vi "Dresden R2R Sputter 03.02.2018 IY24.vi"() -> ()   [LabVIEW 2009] (continued)
                                }
                                }
                                }
                                }
                                frame #4 {
                                n32415 = local read "R Cmb Ch2 Step5 Coating Power Active"() -> (w37013:bool)
                                n32416 = case shown="True" w37013 {
                                frame #0 {
                                }
                                frame #1 {
                                n32417 = stacked-sequence {
                                frame #0 {
                                n32418 = local read "Semi"() -> (w37014:bool)
                                n32419 = case shown="False" w37014 {
                                frame #0 {
                                n32420 = local read "R Cmb Ch3 Step5 Coating Power"() -> (w37016:dbl)
                                n32421 = Wait (ms)(milliseconds to wait=u32 200) -> ()  [unwired: 1 out]
                                n32422 = local write "Set DC Power       : 2"(w37016) -> ()
                                }
                                frame #1 {
                                }
                                }
                                }
                                frame #1 {
                                n32423 = local read "Semi"() -> (w37017:bool)
                                n32424 = case shown="False" w37017 {
                                frame #0 {
                                n32425 = local write "Dc_auto_set"(TRUE ("Dc_auto_set")) -> ()
                                }
                                frame #1 {
                                }
                                }
                                }
                                frame #2 {
                                n32426 = while {
                                stop <- w37023 stop-if-true
                                n32427 = local read "R Cmb Interval length"() -> (w37022:dbl)
                                n32428 = local read "Actual Length"() -> (w37026:dbl)
                                n32429 = Multiply(x=w37022, y=5.0) -> (x*y=w37020:dbl)
                                n32430 = Greater Or Equal?(x=w37026, y=w37020) -> (x >= y?=w37025:bool)
                                n32431 = local read "Semi"() -> (w37024:bool)
                                n32432 = Or(x=w37025, y=w37024) -> (x .or. y?=w37023:bool)
                                n32433 = Wait Until Next ms Multiple(millisecond multiple=u32 300) -> ()  [unwired: 1 out]
                                }
                                }
                                }
                                }
                                }
                                }
                                }
                                }
                                frame #1 {
                                }
                                }
                                }
                                frame #13 {
                                n32434 = local read "Semi"() -> (w37027:bool)
                                n32435 = case shown="False" w37027 {
                                frame #0 {
                                n32436 = local write "SDC1 13b"(TRUE ("SDC1 13b")) -> ()
                                n32437 = Wait (ms)(milliseconds to wait=u32 1000) -> ()  [unwired: 1 out]
                                }
                                frame #1 {
                                }
                                }
                                }
                                }
                                }
                                frame #13 {
                                # "CLOSE DC"
                                n32438 = local read "Semi"() -> (w37030:bool)
                                n32439 = case shown="False" w37030 {
                                frame #0 {
                                n32440 = stacked-sequence {
                                frame #0 {
                                n32441 = local read "Semi"() -> (w37031:bool)
                                n32442 = case shown="False" w37031 {
                                frame #0 {
                                n32443 = local write "Dc_auto_off"(TRUE ("Dc_auto_off")) -> ()
                                }
                                frame #1 {
                                }
                                }
                                }
                                frame #1 {
                                n32444 = local read "Semi"() -> (w37033:bool)
                                n32445 = case shown="False" w37033 {
                                frame #0 {
                                n32446 = Wait (ms)(milliseconds to wait=u32 1000) -> ()  [unwired: 1 out]
                                }
                                frame #1 {
                                }
                                }
                                }
                                frame #2 {
                                n32447 = local read "Semi"() -> (w37035:bool)
                                n32448 = case shown="False" w37035 {
                                frame #0 {
                                n32449 = local write "Dc_auto_set_zero"(TRUE ("Dc_auto_set")) -> ()
                                }
                                frame #1 {
                                }
                                }
                                }
                                frame #3 {
                                n32450 = local read "Semi"() -> (w37037:bool)
                                n32451 = case shown="False" w37037 {
                                frame #0 {
                                n32452 = Wait (ms)(milliseconds to wait=u32 1000) -> ()  [unwired: 1 out]
                                }
                                frame #1 {
                                }
                                }
                                }
                                frame #4 {
                                n32453 = local read "Semi"() -> (w37039:bool)
                                n32454 = case shown="False" w37039 {
                                frame #0 {
                                n32455 = while {
                                i -> [w37051]
                                stop <- w37040 stop-if-true
                                n32456 = Greater?(x=w37051, y=600) -> (0:w37050:bool)
                                n32457 = case shown="True" w37050 {
                                frame #0 {
                                }
                                frame #1 {
                                n32458 = local write "Semi"(TRUE ("Semi")) -> ()
                                n32459 = local write "Error Message"("Sputter Process cancelled.\nPlease Check DC connections." ("Error Message")) -> ()
                                }
                                }
                                n32460 = local read "Actual DC Power : 2"() -> (w37045:dbl)
                                n32461 = local read "Actual DC Volt2"() -> (w37044:dbl)
                                n32462 = Less?(x=w37045, y=10.0) -> (x < y?=w37048:bool)
                                n32463 = Less?(x=w37044, y=20.0) -> (x < y?=w37049:bool)
                                n32464 = And(x=w37048, y=w37049) -> (x .and. y?=w37042:bool)
                                n32465 = local read "Semi"() -> (w37041:bool)
                                n32466 = Wait Until Next ms Multiple(millisecond multiple=u32 500) -> ()  [unwired: 1 out]
                                n32467 = Compound Arithmetic op=OR(w37042, w37041) -> (w37040:bool)
                                }
                                }
                                frame #1 {
                                }
                                }
                                }
                                frame #5 {
                                n32468 = local read "Semi"() -> (w37055:bool)
                                n32469 = case shown="False" w37055 {
                                frame #0 {
                                n32470 = while {
                                i -> [w37061]
                                stop <- w37056 stop-if-true
                                n32471 = Greater?(x=w37061, y=50) -> (0:w37060:bool)
                                n32472 = case shown="True" w37060 {
                                frame #0 {
                                }
                                frame #1 {
                                n32473 = local write "Semi"(TRUE ("Semi")) -> ()
                                n32474 = local write "Error Message"("Sputter Process cancelled.\nPlease Check DCPS-SW2." ("Error Message")) -> ()
                                }
                                }
                                n32475 = local read "Cnt_Dcps_sw2_di"() -> (w37059:bool)
                                n32476 = case shown="True" w37059 {
                                tunnel: [TRUE ("Cnt_Dcps_sw1_do") FALSE ("Cnt_Dcps_sw1_do")] -> w37058
                                frame #0 {
                                }
                                frame #1 {
                                n32477 = local write "Cnt_Dcps_sw2_do"(FALSE ("Cnt_Dcps_sw1_do")) -> ()
                                n32478 = Wait Until Next ms Multiple(millisecond multiple=u32 500) -> ()  [unwired: 1 out]
                                }
                                }
                                n32479 = local read "Semi"() -> (w37057:bool)
                                n32480 = Or(x=w37058, y=w37057) -> (x .or. y?=w37056:bool)
                                }
                                }
                                frame #1 {
                                }
                                }
                                }
                                frame #6 {
                                n32481 = local read "Semi"() -> (w37069:bool)
                                n32482 = case shown="False" w37069 {
                                frame #0 {
                                n32483 = Wait (ms)(milliseconds to wait=u32 1000) -> ()  [unwired: 1 out]
                                n32484 = local write "SDC1 25"(TRUE ("SDC1 25")) -> ()
                                }
                                frame #1 {
                                }
                                }
                                }
                                }
                                }
                                frame #1 {
                                }
                                }
                                }
                                frame #14 {
                                # "PC-BV OPEN"
                                n32485 = stacked-sequence {
                                frame #0 {
                                n32486 = local read "Semi"() -> (w37072:bool)
                                n32487 = case shown="False" w37072 {
                                frame #0 {
                                n32488 = stacked-sequence {
                                frame #0 {
                                n32489 = local read "Semi"() -> (w37073:bool)
                                n32490 = case shown="False" w37073 {
                                frame #0 {
                                n32491 = local write "Pc_bv3_auto_open"(TRUE ("Tp1_auto_start")) -> ()
                                }
                                frame #1 {
                                }
                                }
                                }
                                frame #1 {
                                n32492 = local read "Semi"() -> (w37075:bool)
                                n32493 = case shown="False" w37075 {
                                frame #0 {
                                n32494 = Wait (ms)(milliseconds to wait=u32 1000) -> ()  [unwired: 1 out]
                                }
                                frame #1 {
                                }
                                }
                                }
                                frame #2 {
                                n32495 = local read "Semi"() -> (w37077:bool)
                                n32496 = case shown="False" w37077 {
                                frame #0 {
                                n32497 = while {
                                i -> [w37083]
                                stop <- w37079 stop-if-true
                                n32498 = local read "Pc_bv_opened_ch3"() -> (w37081:bool)
                                n32499 = Greater?(x=w37083, y=120) -> (0:w37082:bool)
                                n32500 = local read "Semi"() -> (w37080:bool)
                                n32501 = Compound Arithmetic op=OR(w37080, w37081, w37082) -> (w37079:bool)
                                n32502 = Wait (ms)(milliseconds to wait=u32 500) -> ()  [unwired: 1 out]
                                }
                                }
                                frame #1 {
                                }
                                }
                                }
                                frame #3 {
                                n32503 = local read "Semi"() -> (w37085:bool)
                                n32504 = case shown="False" w37085 {
                                frame #0 {
                                n32505 = local read "Pc_bv_opened_ch3"() -> (w37086:bool)
                                n32506 = case shown="False" w37086 {
                                frame #0 {
                                n32507 = local write "Pc_bv3_auto_open"(TRUE ("Pc_bv1_auto_open")) -> ()
                                }
                                frame #1 {
                                }
                                }
                                }
                                frame #1 {
                                }
                                }
                                }
                                frame #4 {
                                n32508 = local read "Semi"() -> (w37088:bool)
                                n32509 = case shown="False" w37088 {
                                frame #0 {
                                n32510 = local read "Pc_bv_opened_ch3"() -> (w37089:bool)
                                n32511 = case shown="False" w37089 {
                                frame #0 {
                                n32512 = Wait (ms)(milliseconds to wait=u32 1000) -> ()  [unwired: 1 out]
                                }
                                frame #1 {
                                }
                                }
                                }
                                frame #1 {
                                }
                                }
                                }
                                frame #5 {
                                n32513 = local read "Semi"() -> (w37091:bool)
                                n32514 = case shown="False" w37091 {
                                frame #0 {
                                n32515 = while {
                                i -> [w37097]
                                stop <- w37093 stop-if-true
                                n32516 = local read "Pc_bv_opened_ch3"() -> (w37095:bool)
                                n32517 = Greater?(x=w37097, y=120) -> (0:w37096:bool)
                                n32518 = local read "Semi"() -> (w37094:bool)
                                n32519 = Compound Arithmetic op=OR(w37094, w37095, w37096) -> (w37093:bool)
                                n32520 = Wait (ms)(milliseconds to wait=u32 500) -> ()  [unwired: 1 out]
                                }
                                }
                                frame #1 {
                                }
                                }
                                }
                                frame #6 {
                                n32521 = local read "Semi"() -> (w37099:bool)
                                n32522 = case shown="False" w37099 {
                                frame #0 {
                                n32523 = local read "Pc_bv_opened_ch3"() -> (w37100:bool)
                                n32524 = case shown="False" w37100 {
                                frame #0 {
                                n32525 = local write "Error Message"("Start up process  cancelled\nbecause  PC-BV not opened.\nPlease check PC-BV1 connections." ("Error Message")) -> ()
                                n32526 = Wait (ms)(milliseconds to wait=u32 1000) -> ()  [unwired: 1 out]
                                }
                                frame #1 {
                                }
                                }
                                }
                                frame #1 {
                                }
                                }
                                }
                                }
                                }
                                frame #1 {
                                }
                                }
                                }
                                frame #1 {
                                n32527 = local read "Semi"() -> (w37103:bool)
                                n32528 = case shown="False" w37103 {
                                frame #0 {
                                n32529 = Wait (ms)(milliseconds to wait=u32 1000) -> ()  [unwired: 1 out]
                                n32530 = local write "SDC1 28"(TRUE ("SDC1 28")) -> ()
                                }
                                frame #1 {
                                }
                                }
                                }
                                }
                                }
                                frame #15 {
                                # "set ar zero"
                                n32531 = stacked-sequence {
                                frame #0 {
                                n32532 = local read "Semi"() -> (w37106:bool)
                                n32533 = case shown="False" w37106 {
                                frame #0 {
                                n32534 = stacked-sequence {
                                frame #0 {
                                n32535 = local read "Semi"() -> (w37107:bool)
                                n32536 = case shown="False" w37107 {
                                frame #0 {
                                n32537 = local write "Ar_auto_set_zero_ch3"(TRUE ("Ar_auto_set_zero_ch1")) -> ()
                                }
                                frame #1 {
                                }
                                }
                                }
                                frame #1 {
                                n32538 = local read "Semi"() -> (w37109:bool)
                                n32539 = case shown="False" w37109 {
                                frame #0 {
                                n32540 = while {
                                i -> [w37112]
                                stop <- w37111 stop-if-true
                                n32541 = Greater?(x=w37112, y=150) -> (0:w37111:bool)
                                n32542 = local read "Semi"() -> (w37110:bool)
                                n32543 = case shown="False" w37110 {
                                tunnel: [FALSE TRUE] -> _
                                frame #0 {
                                n32544 = Wait Until Next ms Multiple(millisecond multiple=u32 200) -> ()  [unwired: 1 out]
                                }
                                frame #1 {
                                }
                                }
                                }
                                }
                                frame #1 {
                                }
                                }
                                }
                                frame #2 {
                                n32545 = local read "Semi"() -> (w37117:bool)
                                n32546 = case shown="False" w37117 {
                                frame #0 {
                                n32547 = local read "Ar_sccm_act 2"() -> (w37118:dbl)
                                n32548 = Less?(x=w37118, y=1) -> (x < y?=w37119:bool)
                                n32549 = case shown="False" w37119 {
                                frame #0 {
                                n32550 = local write "Ar_auto_set_zero_ch3"(TRUE ("Ar_auto_set_zero_ch1")) -> ()
                                }
                                frame #1 {
                                }
                                }
                                }
                                frame #1 {
                                }
                                }
                                }
                                frame #3 {
                                n32551 = local read "Semi"() -> (w37122:bool)
                                n32552 = case shown="False" w37122 {
                                frame #0 {
                                n32553 = local read "Ar_sccm_act 2"() -> (w37123:dbl)
                                n32554 = Less?(x=w37123, y=1) -> (x < y?=w37124:bool)
                                n32555 = case shown="False" w37124 {
                                frame #0 {
                                n32556 = while {
                                i -> [w37130]
                                stop <- w37127 stop-if-true
                                n32557 = Greater?(x=w37130, y=150) -> (0:w37128:bool)
                                n32558 = local read "Semi"() -> (w37126:bool)
                                n32559 = case shown="True" w37126 {
                                tunnel: [FALSE FALSE] -> w37129
                                frame #0 {
                                }
                                frame #1 {
                                n32560 = Wait Until Next ms Multiple(millisecond multiple=u32 200) -> ()  [unwired: 1 out]
                                }
                                }
                                n32561 = Or(x=w37129, y=w37128) -> (x .or. y?=w37127:bool)
                                }
                                }
                                frame #1 {
                                }
                                }
                                }
                                frame #1 {
                                }
                                }
                                }
                                frame #4 {
                                n32562 = local read "Semi"() -> (w37135:bool)
                                n32563 = case shown="False" w37135 {
                                frame #0 {
                                n32564 = Wait (ms)(milliseconds to wait=u32 1000) -> ()  [unwired: 1 out]
                                }
                                frame #1 {
                                }
                                }
                                }
                                }
                                }
                                frame #1 {
                                }
                                }
                                }
                                frame #1 {
                                n32565 = local read "Semi"() -> (w37137:bool)
                                n32566 = case shown="False" w37137 {
                                frame #0 {
                                n32567 = local write "SDC1 26"(TRUE ("SDC1 26")) -> ()
                                n32568 = Wait (ms)(milliseconds to wait=u32 1000) -> ()  [unwired: 1 out]
                                }
                                frame #1 {
                                }
                                }
                                }
                                }
                                }
                                frame #16 {
                                # "sov-ar close"
                                n32569 = stacked-sequence {
                                frame #0 {
                                n32570 = local read "Semi"() -> (w37140:bool)
                                n32571 = case shown="False" w37140 {
                                frame #0 {
                                n32572 = while {
                                i -> [w37146]
                                stop <- w37141 stop-if-true
                                n32573 = Greater?(x=w37146, y=50) -> (0:w37145:bool)
                                n32574 = case shown="True" w37145 {
                                frame #0 {
                                }
                                frame #1 {
                                n32575 = local write "Semi"(TRUE ("Semi")) -> ()
                                n32576 = local write "Error Message"("Coating Process  \nwas cancelled.\nPlease check \nSOV-Ar connection." ("Error Message")) -> ()
                                }
                                }
                                n32577 = local read "Ch3_Sov_Ar_di"() -> (w37144:bool)
                                n32578 = case shown="True" w37144 {
                                tunnel: [TRUE FALSE] -> w37143
                                frame #0 {
                                }
                                frame #1 {
                                n32579 = local write "Ch3_Sov_Ar_do"(FALSE ("Ch1_WFC_do")) -> ()
                                n32580 = Wait Until Next ms Multiple(millisecond multiple=u32 200) -> ()  [unwired: 1 out]
                                }
                                }
                                n32581 = local read "Semi"() -> (w37142:bool)
                                n32582 = Or(x=w37143, y=w37142) -> (x .or. y?=w37141:bool)
                                }
                                }
                                frame #1 {
                                }
                                }
                                }
                                frame #1 {
                                n32583 = local read "Semi"() -> (w37154:bool)
                                n32584 = case shown="False" w37154 {
                                frame #0 {
                                n32585 = local write "SDC1 27"(TRUE ("SDC1 27")) -> ()
                                n32586 = Wait (ms)(milliseconds to wait=u32 1000) -> ()  [unwired: 1 out]
                                }
                                frame #1 {
                                }
                                }
                                }
                                }
                                }
                                frame #17 {
                                # "CC OPEN"
                                n32587 = stacked-sequence {
                                frame #0 {
                                n32588 = local read "Semi"() -> (w37157:bool)
                                n32589 = case shown="False" w37157 {
                                frame #0 {
                                n32590 = while {
                                i -> [w37163]
                                stop <- w37158 stop-if-true
                                n32591 = Greater?(x=w37163, y=50) -> (0:w37162:bool)
                                n32592 = case shown="True" w37162 {
                                frame #0 {
                                }
                                frame #1 {
                                n32593 = local write "Semi"(TRUE ("Semi")) -> ()
                                n32594 = local write "Error Message"("Coating Process  \nwas cancelled.\nPlease check \nBG-BV connection." ("Error Message")) -> ()
                                }
                                }
                                n32595 = local read "Ch3_Cc_on_off_di"() -> (w37161:bool)
                                n32596 = case shown="False" w37161 {
                                tunnel: [FALSE TRUE] -> w37160
                                frame #0 {
                                n32597 = local write "Ch3_Cc_on_off_do"(TRUE ("Ch1_WFC_do")) -> ()
                                n32598 = Wait Until Next ms Multiple(millisecond multiple=u32 200) -> ()  [unwired: 1 out]
                                }
                                frame #1 {
                                }
                                }
                                n32599 = local read "Semi"() -> (w37159:bool)
                                n32600 = Or(x=w37160, y=w37159) -> (x .or. y?=w37158:bool)
                                }
                                }
                                frame #1 {
                                }
                                }
                                }
                                frame #1 {
                                n32601 = local read "Semi"() -> (w37171:bool)
                                n32602 = case shown="False" w37171 {
                                frame #0 {
                                n32603 = while {
                                i -> [w37176]
                                stop <- w37174 stop-if-true
                                n32604 = Greater?(x=w37176, y=30) -> (0:w37172:bool)
                                n32605 = Wait Until Next ms Multiple(millisecond multiple=u32 1000) -> ()  [unwired: 1 out]
                                n32606 = local read "Semi"() -> (w37175:bool)
                                n32607 = Or(x=w37172, y=w37175) -> (x .or. y?=w37174:bool)
                                }
                                }
                                frame #1 {
                                }
                                }
                                }
                                frame #2 {
                                n32608 = local read "Semi"() -> (w37178:bool)
                                n32609 = case shown="False" w37178 {
                                frame #0 {
                                n32610 = local write "SDC1 27b"(TRUE ("SDC1 3")) -> ()
                                n32611 = Wait (ms)(milliseconds to wait=u32 1000) -> ()  [unwired: 1 out]
                                }
                                frame #1 {
                                }
                                }
                                }
                                }
                                }
                                frame #18 {
                                # "CHECK CHAMBER PRESSURE"
                                n32612 = stacked-sequence {
                                frame #0 {
                                n32613 = local read "Semi"() -> (w37181:bool)
                                n32614 = case shown="False" w37181 {
                                frame #0 {
                                n32615 = while {
                                i -> [w37189]
                                stop <- w37183 stop-if-true
                                n32616 = Greater?(x=w37189, y=300) -> (0:w37188:bool)
                                n32617 = case shown="True" w37188 {
                                frame #0 {
                                }
                                frame #1 {
                                n32618 = local write "Semi"(TRUE ("Semi")) -> ()
                                n32619 = local write "Error Message"("Coating Process cancelled.\nPlease check chamber \nconnections." ("Error Message")) -> ()
                                }
                                }
                                n32620 = local read "Ch_CC_press_ch3 2"() -> (w37182:dbl)
                                n32621 = Greater Or Equal?(x=w37182, y=5e-05 ("CHAMBER PRESSURE 6")) -> (x >= y?=w37186:bool)
                                n32622 = case shown="True" w37186 {
                                tunnel: [TRUE FALSE] -> w37185
                                frame #0 {
                                }
                                frame #1 {
                                n32623 = Wait Until Next ms Multiple(millisecond multiple=u32 200) -> ()  [unwired: 1 out]
                                }
                                }
                                n32624 = local read "Semi"() -> (w37184:bool)
                                n32625 = Or(x=w37185, y=w37184) -> (x .or. y?=w37183:bool)
                                }
                                }
                                frame #1 {
                                }
                                }
                                }
                                frame #1 {
                                n32626 = local read "Semi"() -> (w37196:bool)
                                n32627 = case shown="False" w37196 {
                                frame #0 {
                                n32628 = Wait (ms)(milliseconds to wait=u32 1000) -> ()  [unwired: 1 out]
                                n32629 = local write "SDC1 27c"(TRUE ("SDC1 10")) -> ()
                                }
                                frame #1 {
                                }
                                }
                                }
                                }
                                }
                                frame #19 {
                                # "encoder info  add to other web selection"
                                n32630 = stacked-sequence {
                                frame #0 {
                                n32631 = local read "Semi"() -> (w37199:bool)
                                n32632 = case shown="False" w37199 {
                                frame #0 {
                                # "TC -ROLL"
                                n32633 = local read "Semi"() -> (w37200:bool)
                                n32634 = case shown="False" w37200 {
                                frame #0 {
                                n32635 = stacked-sequence {
                                frame #0 {
                                n32636 = local read "R Web speed(cm/min)"() -> (w37203:dbl)
                                n32637 = local read "R Maximum diameter"() -> (w37201:dbl)
                                n32638 = local read "R Web thicness"() -> (w37202:dbl)
                                n32639 = local write "Change_Max Diameter"(w37201) -> ()
                                n32640 = Wait (ms)(milliseconds to wait=u32 100) -> ()  [unwired: 1 out]
                                n32641 = local write "Web Thickness"(w37202) -> ()
                                n32642 = local write "Web Speed"(w37203) -> ()
                                }
                                frame #1 {
                                n32643 = local write "Calculate 3"(TRUE ("Calculate 3")) -> ()
                                }
                                frame #2 {
                                n32644 = local read "R Cmb Ch2 Step1 Coating Power Active"() -> (w37207:bool)
                                n32645 = local read "R Cmb Ch2 Step2 Coating Power Active"() -> (w37208:bool)
                                n32646 = local read "R Cmb Ch2 Step3 Coating Power Active"() -> (w37209:bool)
                                n32647 = local read "R Cmb Ch2 Step4 Coating Power Active"() -> (w37210:bool)
                                n32648 = local read "R Cmb Ch2 Step5 Coating Power Active"() -> (w37211:bool)
                                n32649 = Boolean To (0,1)(Boolean=w37207) -> (0, 1=w37212:i16)
                                n32650 = Boolean To (0,1)(Boolean=w37208) -> (0, 1=w37213:i16)
                                n32651 = Boolean To (0,1)(Boolean=w37209) -> (0, 1=w37214:i16)
                                n32652 = Boolean To (0,1)(Boolean=w37210) -> (0, 1=w37215:i16)
                                n32653 = Boolean To (0,1)(Boolean=w37211) -> (0, 1=w37216:i16)
                                n32654 = Compound Arithmetic op=ADD(w37212, w37213, w37214, w37215, w37216) -> (w37218:i16)
                                n32655 = local read "R Cmb Interval length"() -> (w37217:dbl)
                                n32656 = Wait (ms)(milliseconds to wait=u32 200) -> ()  [unwired: 1 out]
                                n32657 = Multiply(x=w37217, y=w37218) -> (x*y=w37219:dbl)
                                n32658 = local write "Total length"(w37219) -> ()
                                }
                                frame #3 {
                                n32659 = Wait (ms)(milliseconds to wait=u32 1000) -> ()  [unwired: 1 out]
                                }
                                frame #4 {
                                n32660 = local read "Change_Max Diameter"() -> (w37222:dbl)
                                n32661 = Wait (ms)(milliseconds to wait=u32 200) -> ()  [unwired: 1 out]
                                n32662 = local write "Initial Min Diameter"(w37222) -> ()
                                }
                                frame #5 {
                                n32663 = local write "Calculate 2"(TRUE ("Calculate_auto")) -> ()
                                }
                                frame #6 {
                                n32664 = local write "Roll_side_select"(enum32{"Left to Right", "Right to Left"}."Right to Left" ("Roll_side_select")) -> ()
                                }
                                frame #7 {
                                n32665 = Wait (ms)(milliseconds to wait=u32 100) -> ()  [unwired: 1 out]
                                n32666 = local write "Parameters_auto_set"(TRUE ("Parameters_auto_set")) -> ()
                                }
                                frame #8 {
                                n32667 = while {
                                i -> [w37231]
                                stop <- w37227 stop-if-true
                                n32668 = Wait Until Next ms Multiple(millisecond multiple=u32 300) -> ()  [unwired: 1 out]
                                n32669 = Greater?(x=w37231, y=100) -> (0:w37228:bool)
                                n32670 = local read "Parameters_auto_set"() -> (w37232:bool)
                                n32671 = case shown="False" w37232 {
                                tunnel: [TRUE FALSE] -> w37229
                                frame #0 {
                                }
                                frame #1 {
                                }
                                }
                                n32672 = Or(x=w37229, y=w37228) -> (x .or. y?=w37227:bool)
                                }
                                }
                                frame #9 {
                                n32673 = local read "R Tension Value"() -> (w37236:dbl)
                                n32674 = Wait (ms)(milliseconds to wait=u32 200) -> ()  [unwired: 1 out]
                                n32675 = local write "TC2_set_value"(w37236) -> ()
                                }
                                frame #10 {
                                n32676 = local write "TC2_auto_set"(TRUE ("TC1_auto_set")) -> ()
                                }
                                frame #11 {
                                w37239 = u16 2 items=["1", "2", "3", "4"] ("Target Chamber Sensor")
                                n32677 = local write "Target Chamber Sensor"(w37239) -> ()
                                }
                                frame #12 {
                                n32678 = local read "Total length"() -> (w37240:dbl)
                                n32679 = local write "Region"(w37240) -> ()
                                }
                                frame #13 {
                                n32680 = local read "Semi"() -> (w37241:bool)
                                n32681 = case shown="False" w37241 {
                                frame #0 {
                                n32682 = local write "Start_roll"(TRUE ("Start_roll")) -> ()
                                n32683 = Wait (ms)(milliseconds to wait=u32 300) -> ()  [unwired: 1 out]
                                }
                                frame #1 {
                                }
                                }
                                }
                                frame #14 {
                                n32684 = local read "Semi"() -> (w37244:bool)
                                n32685 = case shown="False" w37244 {
                                frame #0 {
                                n32686 = while {
                                stop <- w37248 stop-if-true
                                n32687 = Wait Until Next ms Multiple(millisecond multiple=u32 200 ("milliseconds to wait")) -> ()  [unwired: 1 out]
                                n32688 = local read "Start_roll"() -> (w37246:bool)
                                n32689 = Not(x=w37246) -> (.not. x?=w37245:bool)
                                n32690 = local read "Semi"() -> (w37249:bool)
                                n32691 = Or(x=w37245, y=w37249) -> (x .or. y?=w37248:bool)
                                }
                                }
                                frame #1 {
                                }
                                }
                                }
                                }
                                }
                                frame #1 {
                                }
                                }
                                }
                                frame #1 {
                                }
                                }
                                }
                                frame #1 {
                                n32692 = local read "Semi"() -> (w37250:bool)
                                n32693 = case shown="False" w37250 {
                                frame #0 {
                                n32694 = Wait (ms)(milliseconds to wait=u32 1000) -> ()  [unwired: 1 out]
                                n32695 = local write "SDC1 29"(TRUE ("SDC1 29")) -> ()
                                }
                                frame #1 {
                                }
                                }
                                }
                                }
                                }
                                frame #20 {
                                n32696 = local read "Semi"() -> (w37253:bool)
                                n32697 = case shown="False" w37253 {
                                frame #0 {
                                n32698 = Wait (ms)(milliseconds to wait=u32 2500) -> ()  [unwired: 1 out]
                                n32699 = local write "SDC1 30"(TRUE ("SDC1 30")) -> ()
                                n32700 = local write "Cnt_Do_Buzzer"(TRUE ("SDC1 30")) -> ()
                                }
                                frame #1 {
                                }
                                }
                                }
                                frame #21 {
                                n32701 = local read "Semi"() -> (w37257:bool)
                                n32702 = case shown="False" w37257 {
                                frame #0 {
                                n32703 = Wait (ms)(milliseconds to wait=u32 1000) -> ()  [unwired: 1 out]
                                n32704 = local write "Cnt_Do_Buzzer"(FALSE ("SDC1 30")) -> ()
                                }
                                frame #1 {
                                }
                                }
                                }
                                }
                                }
                                frame #1 {
                                }
                                }
                                }
                                }
                                }
                                frame #1 {
                                }
                              }
                            }
                          }
                        }
                      }
                    }
                  }
                }
              }
            }
          }
          "Recipe_number" <- w29428
        }
      }
    }
  }
